vi "Main.vi"() -> ()   [LabVIEW 2018] (continued)
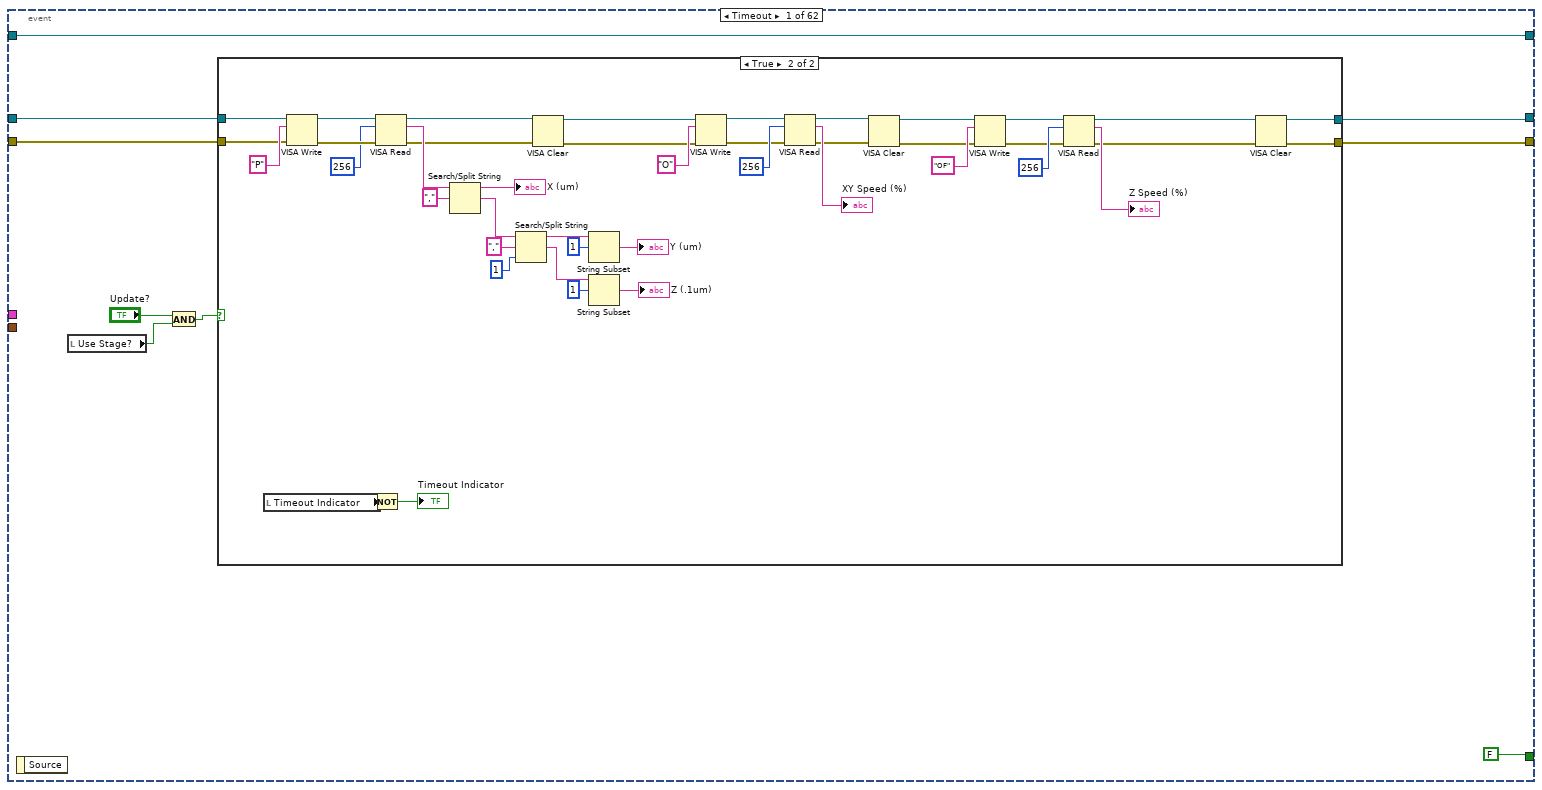
[diagram p4: hidden frame]
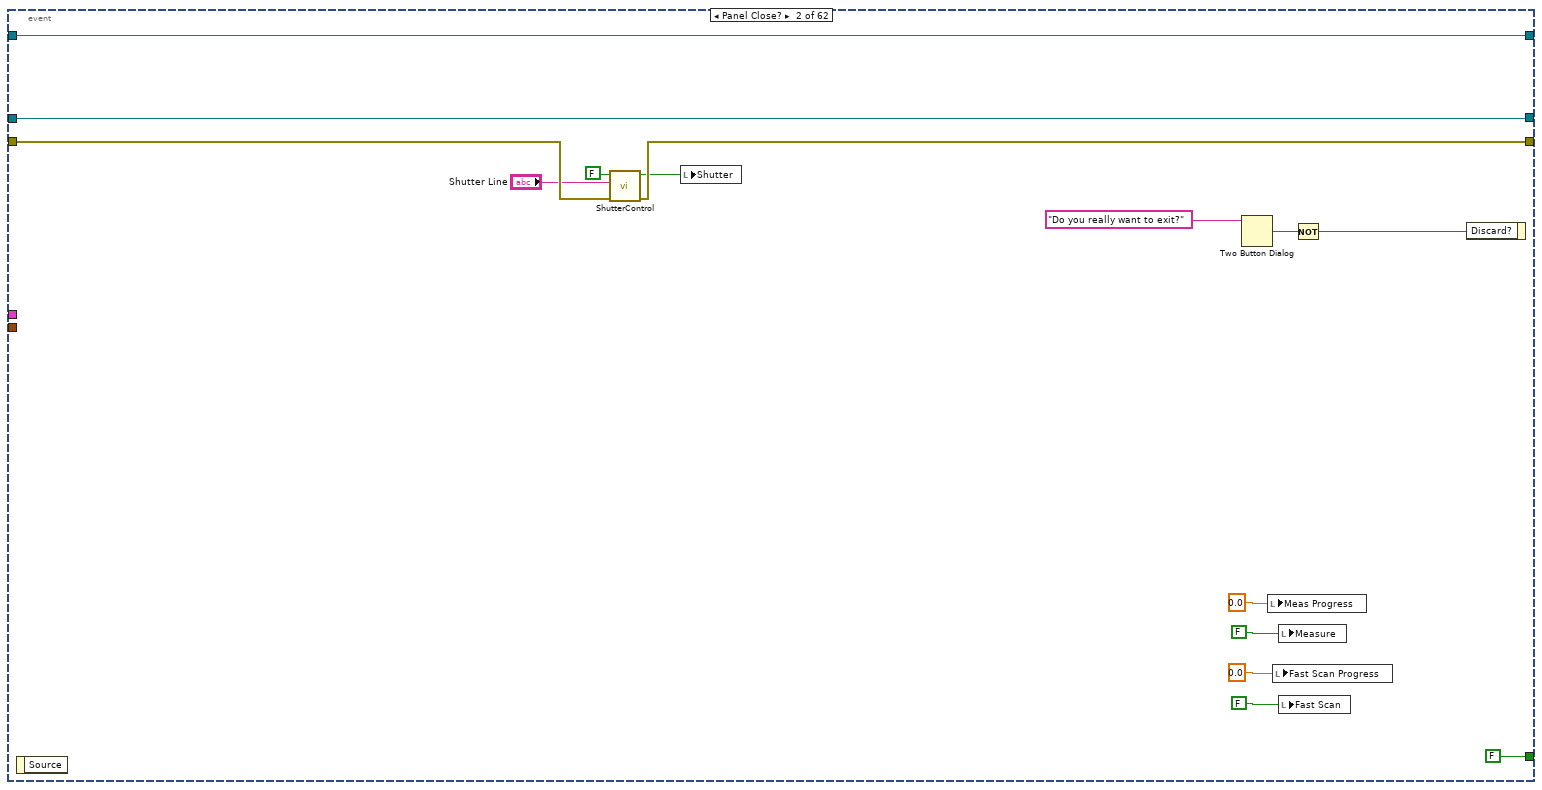
[diagram p6: hidden frame]
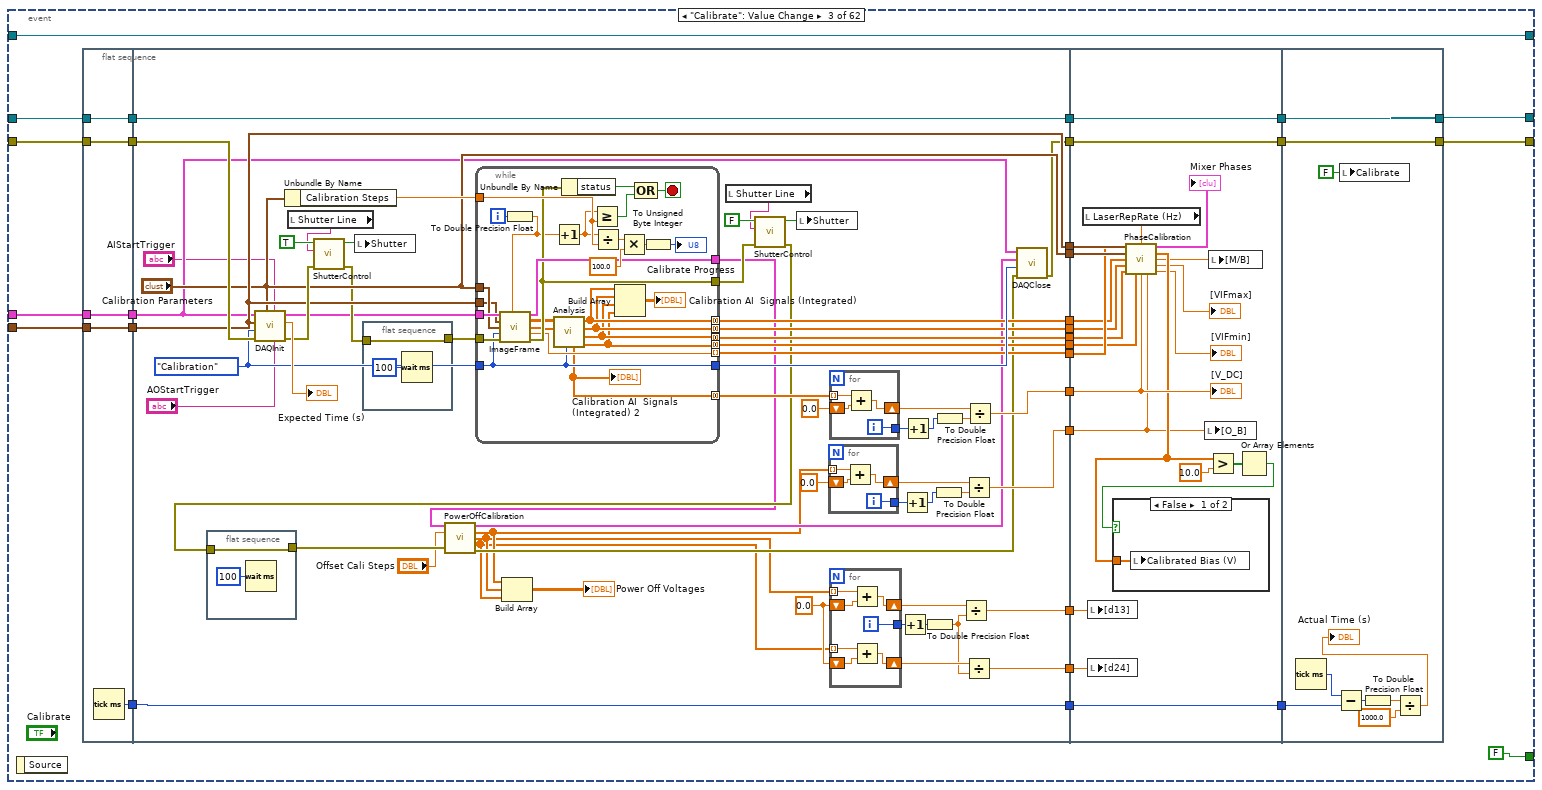
[diagram p7: hidden frame]
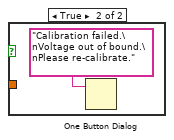
[diagram p8: hidden frame]
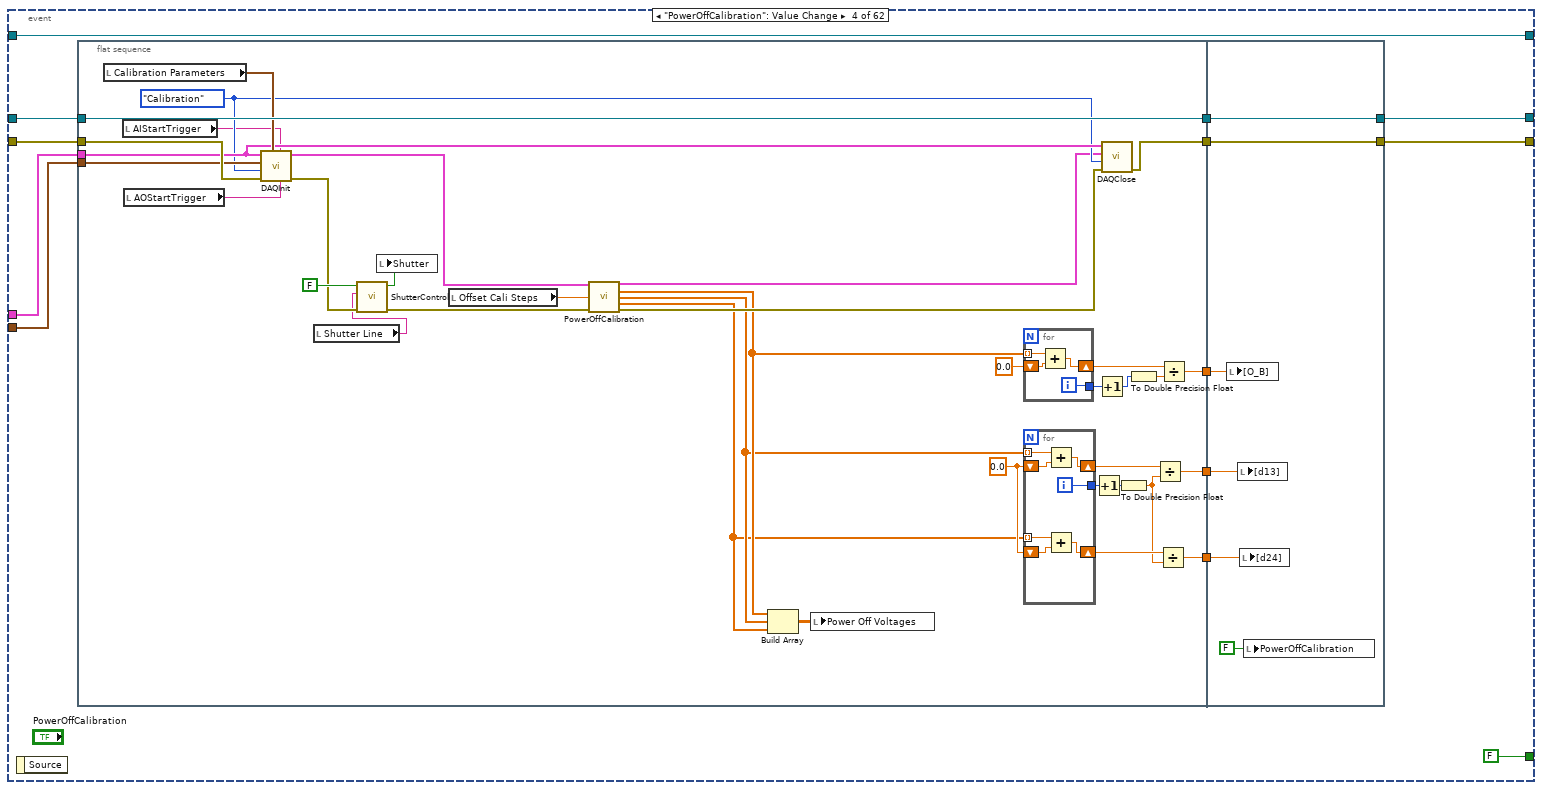
[diagram p9: hidden frame]
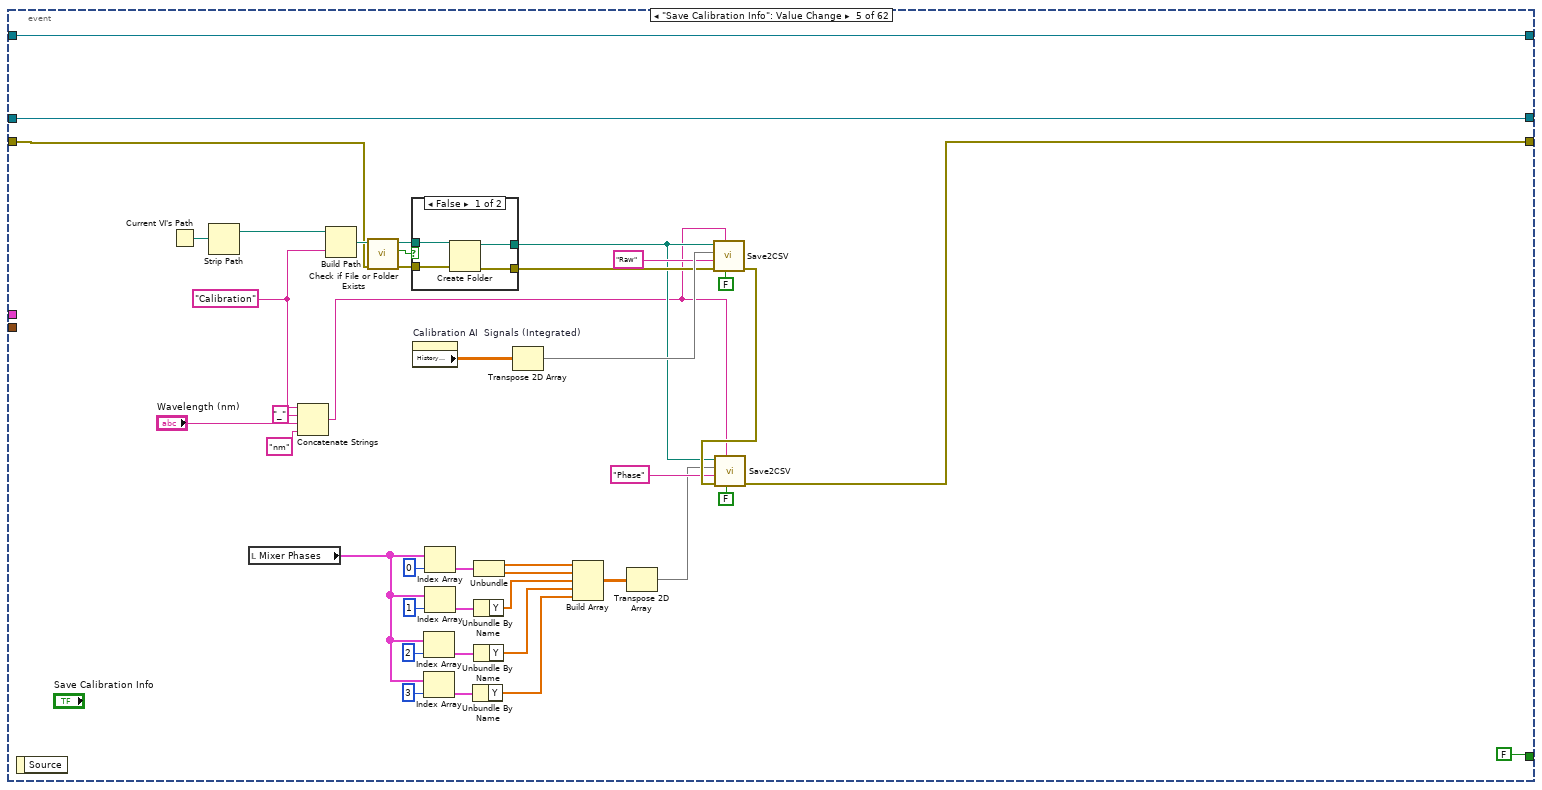
[diagram p10: hidden frame]
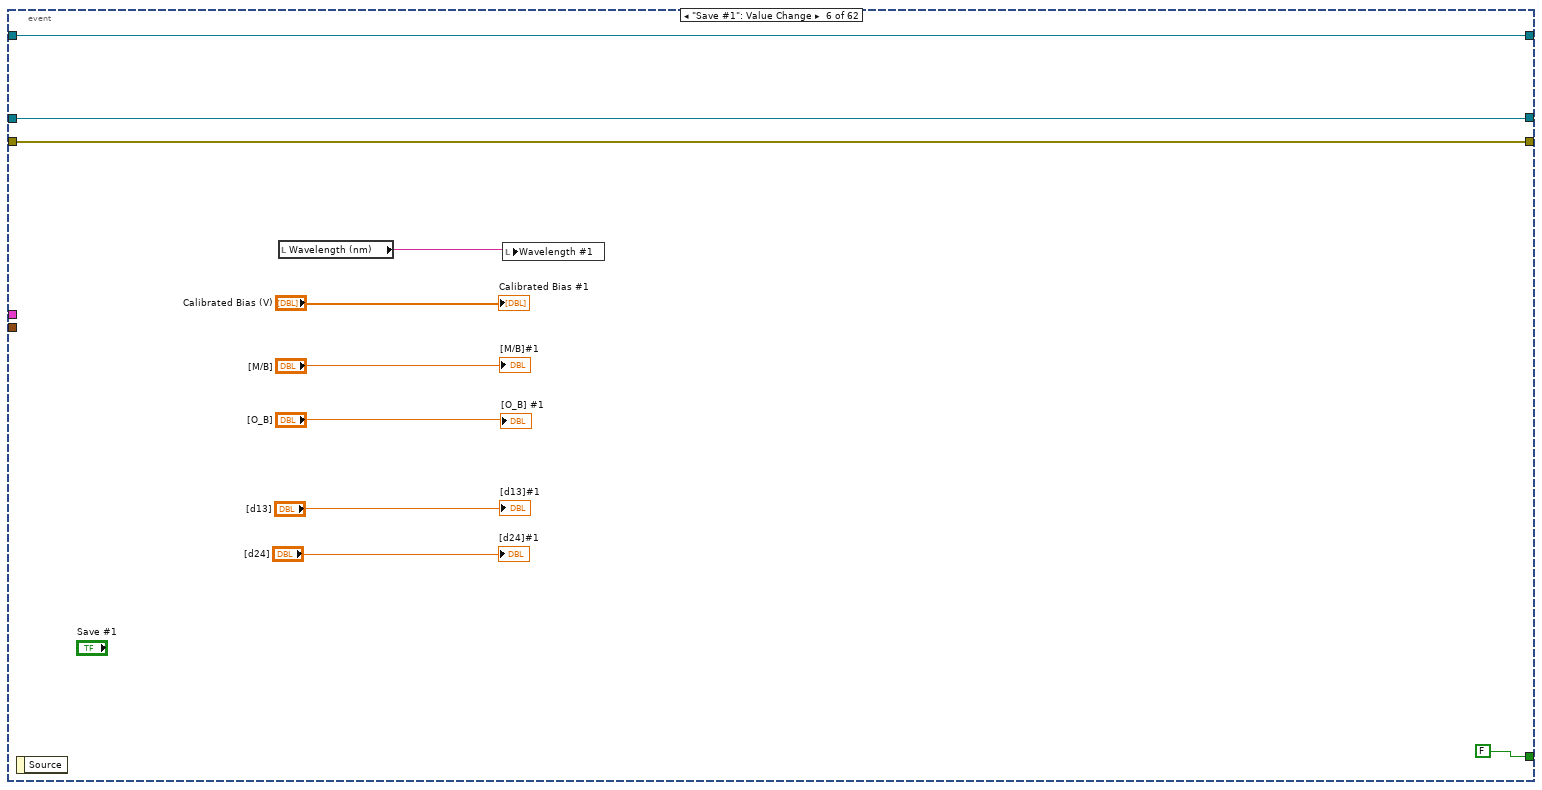
[diagram p12: hidden frame]
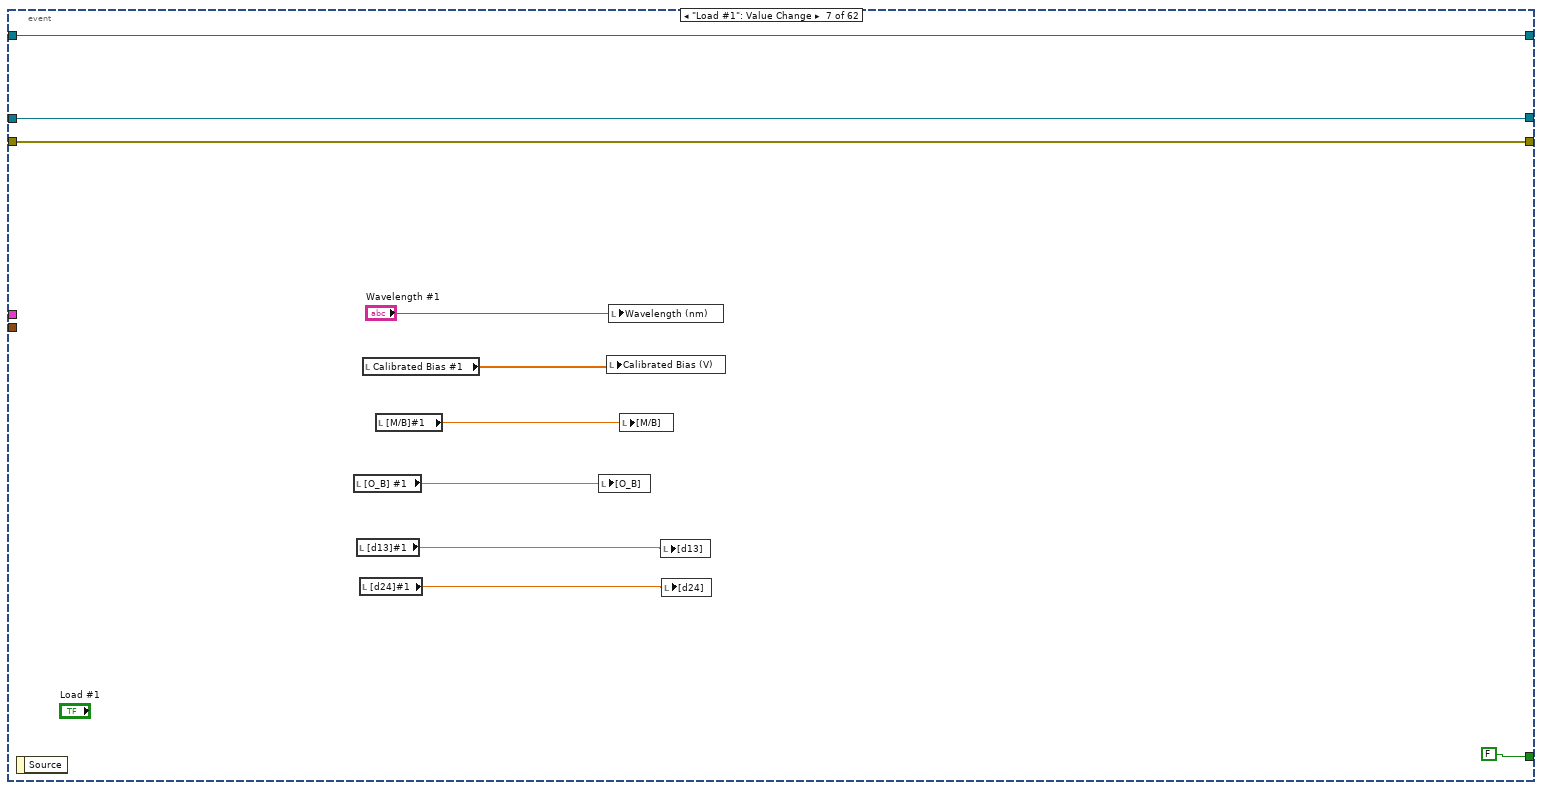
[diagram p13: hidden frame]
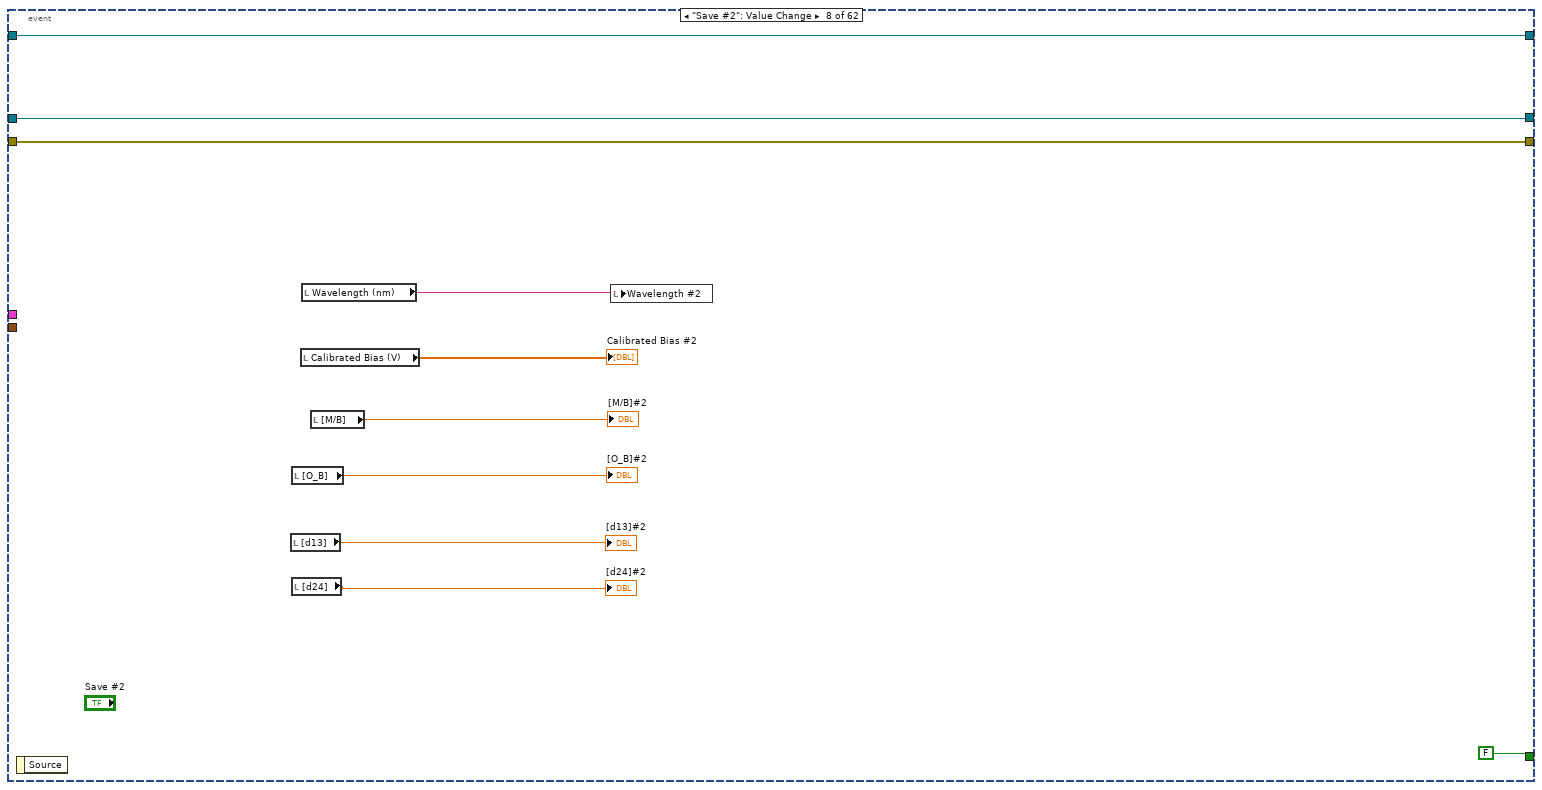
[diagram p14: hidden frame]
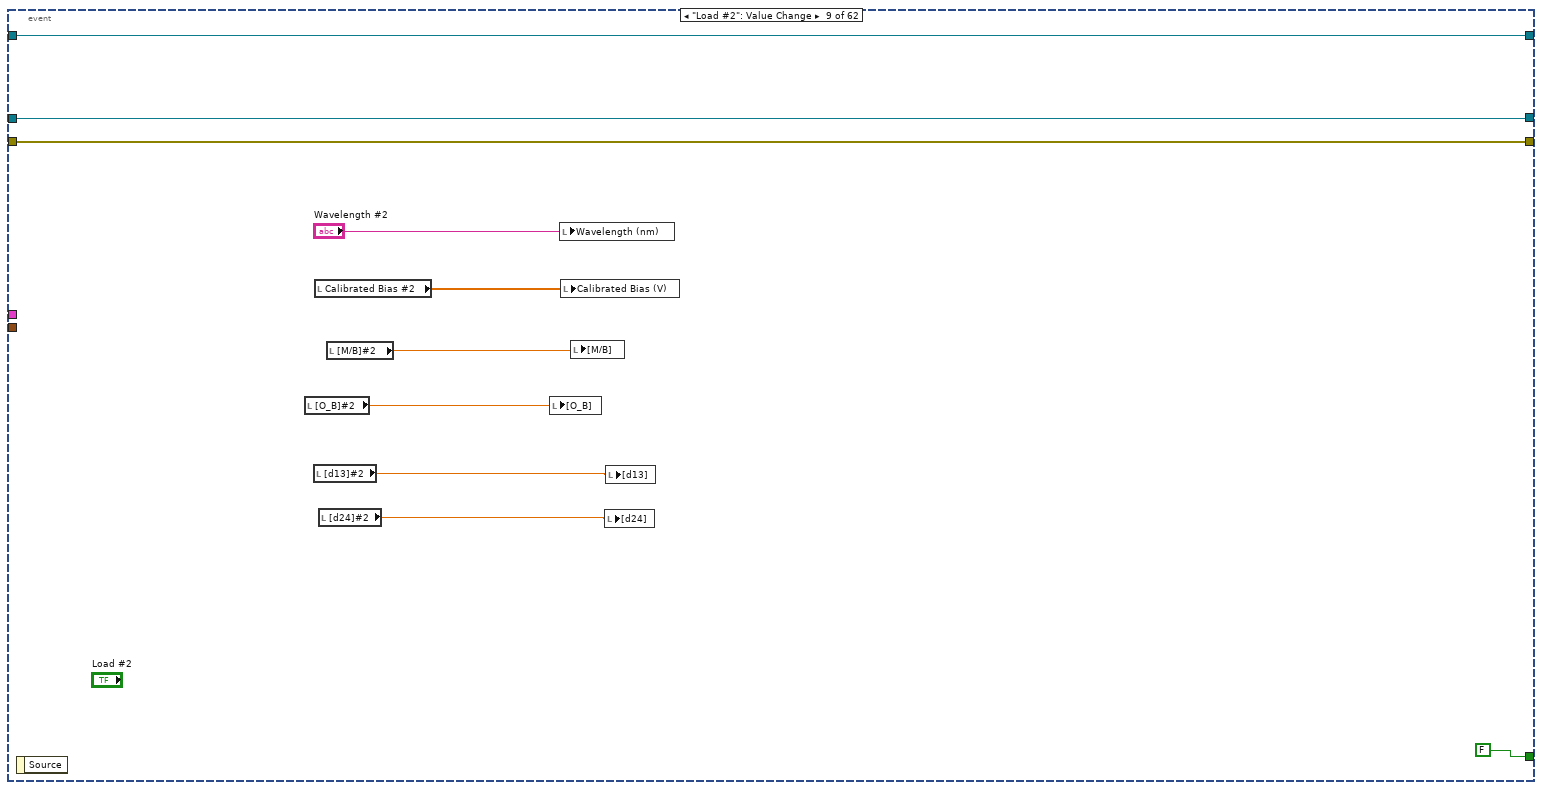
[diagram p15: hidden frame]
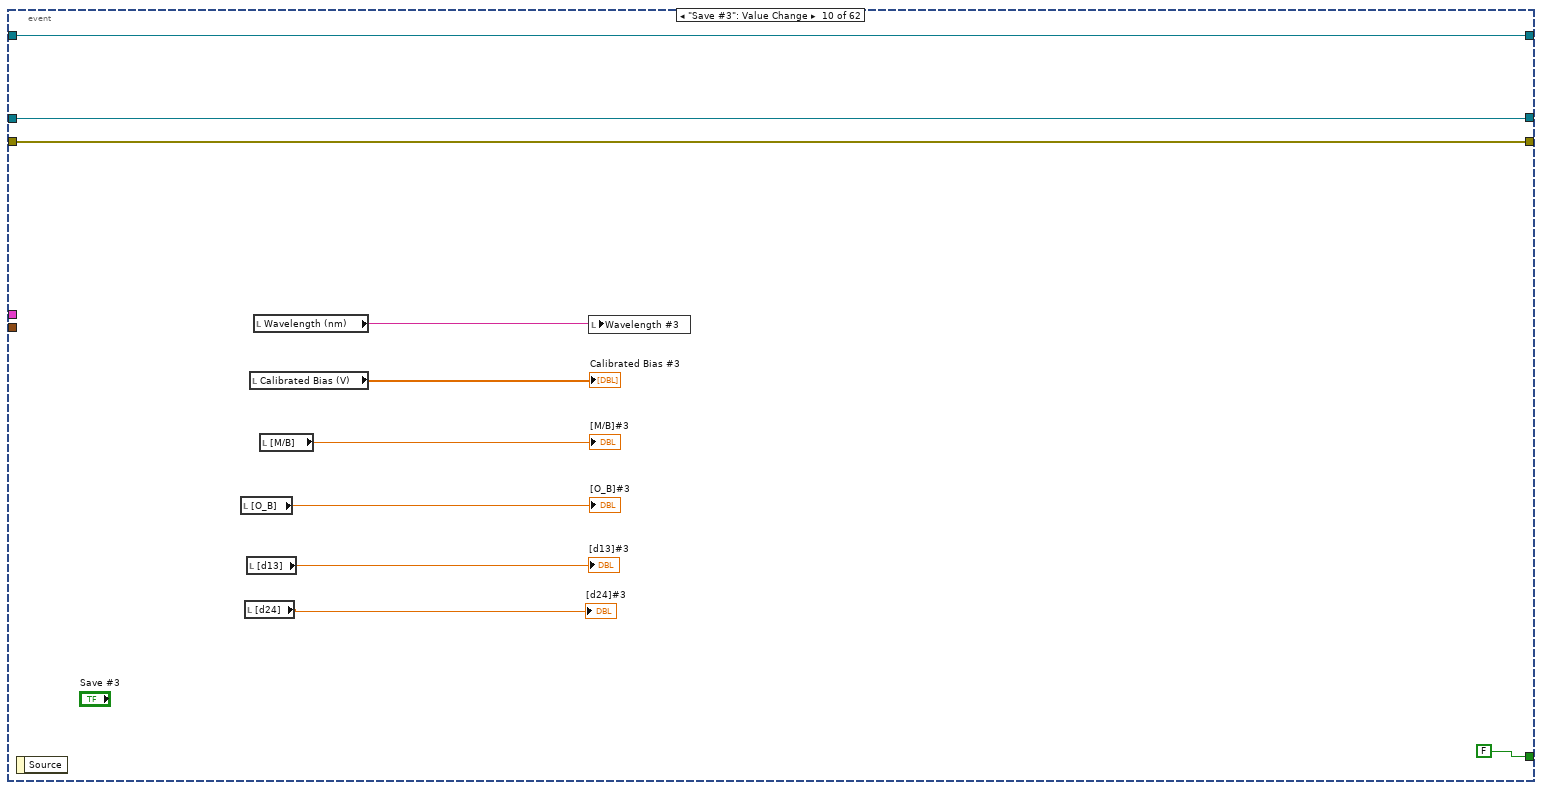
[diagram p16: hidden frame]
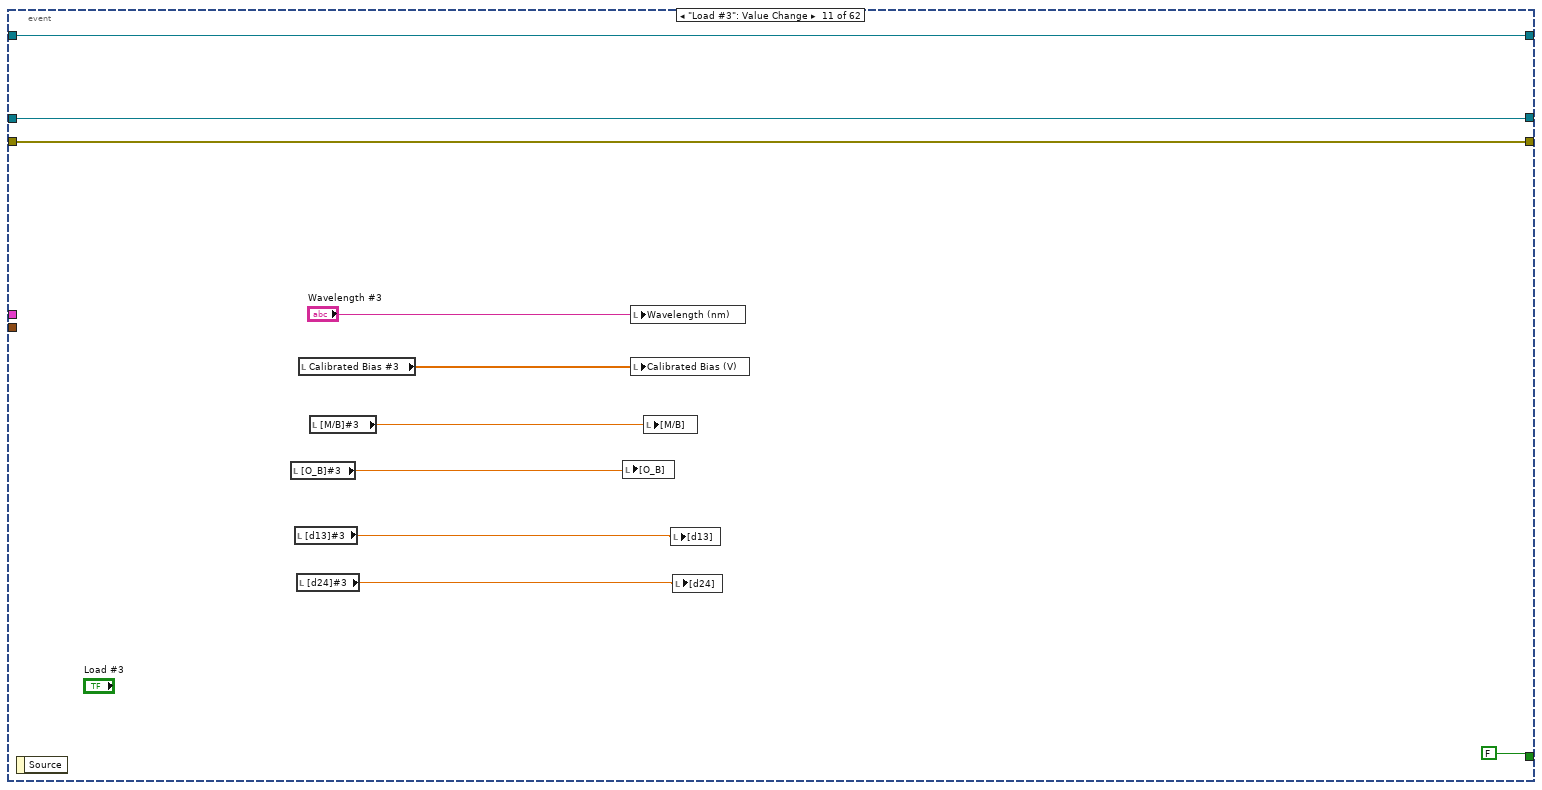
[diagram p17: hidden frame]
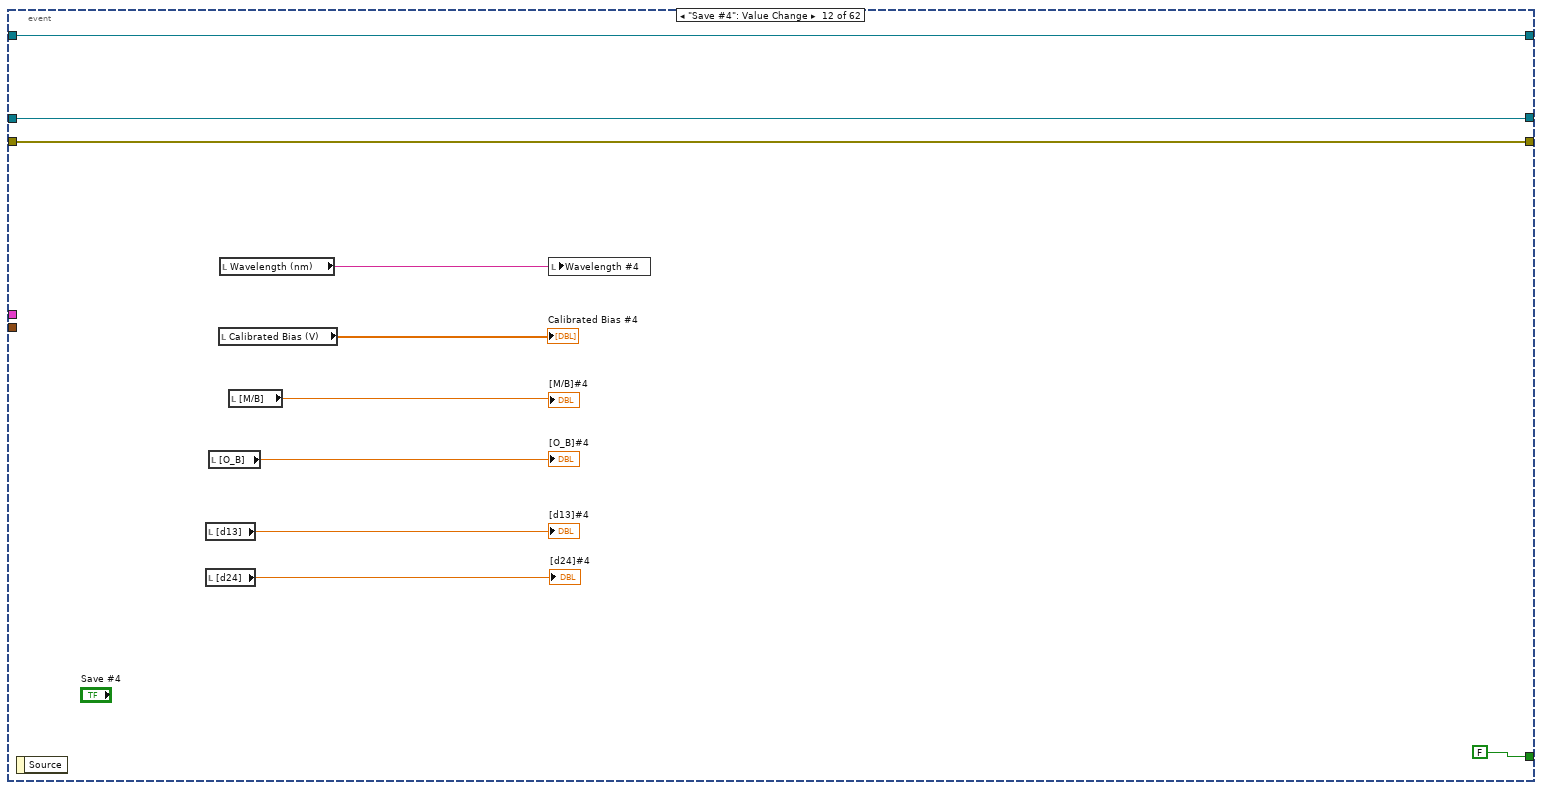
[diagram p18: hidden frame]
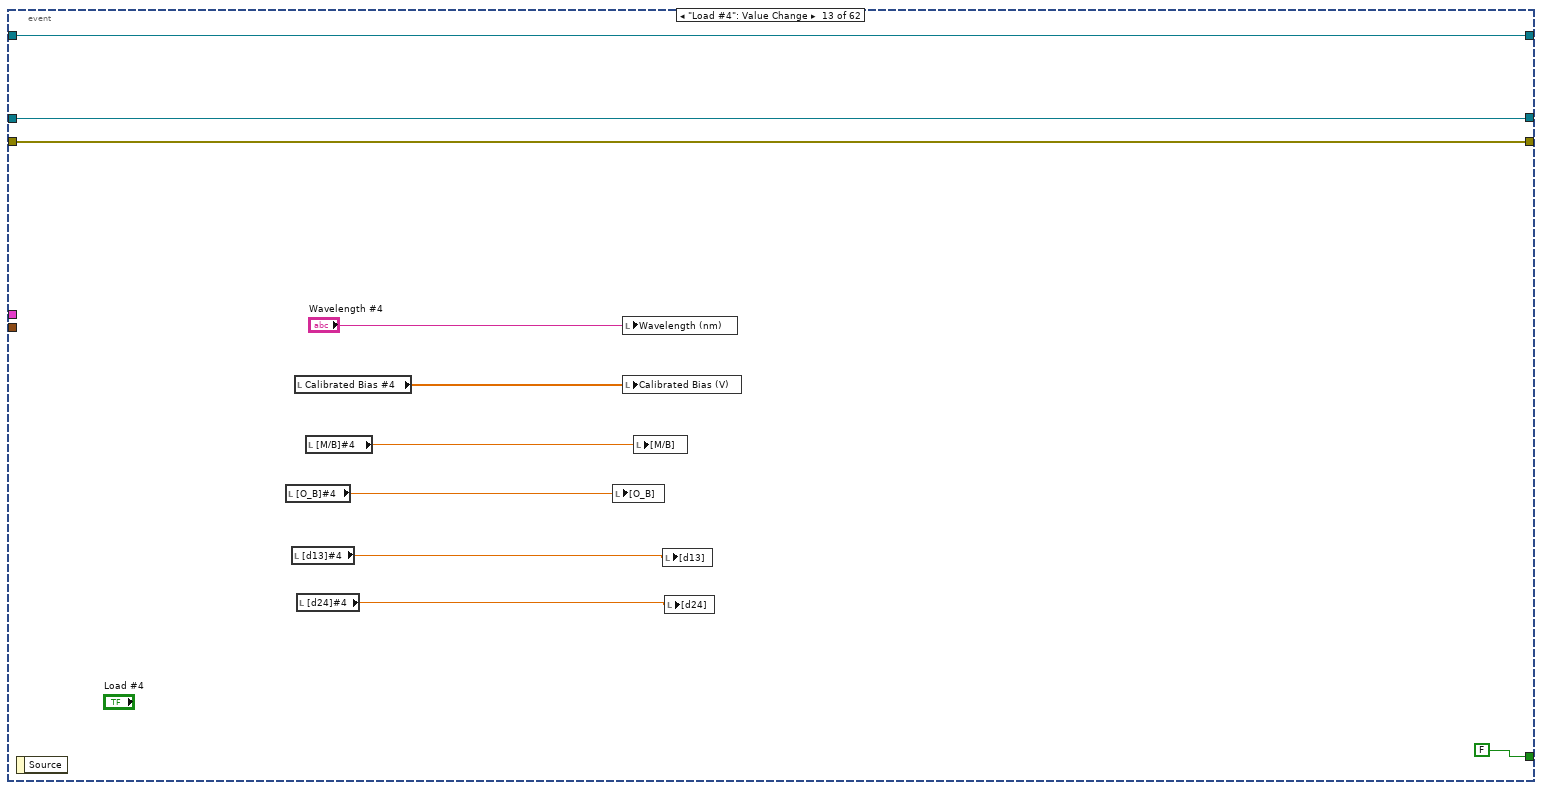
[diagram p19: hidden frame]
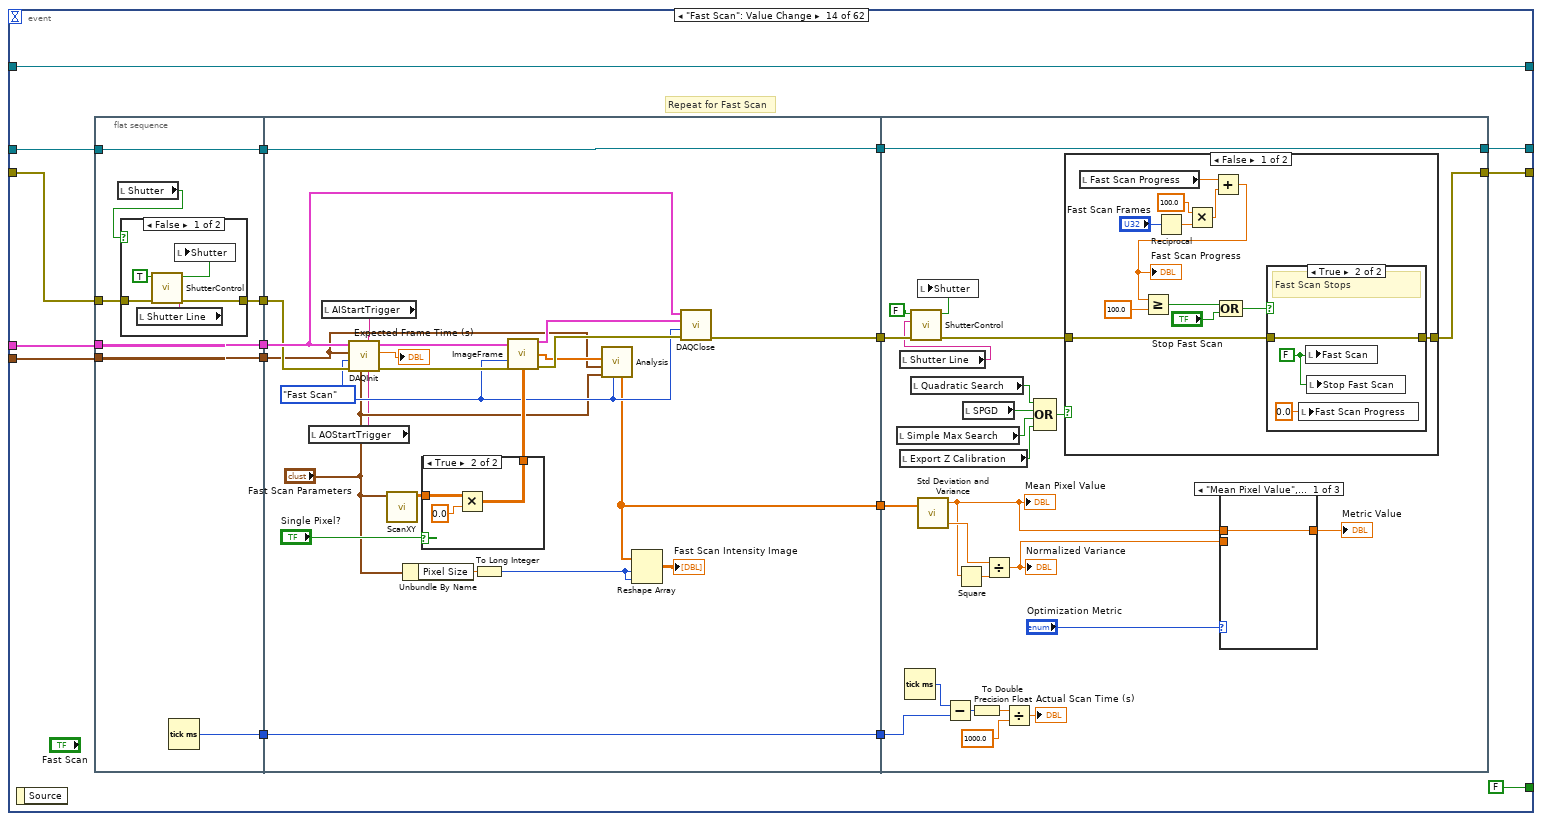
[diagram p20: hidden frame]
          }
        }
      }
      event "Set Current XY to 0": Value Change {
        n1487 = event-data() -> ()  [unwired: 1 in, 1 out]
        n1488 = local read "Use Stage?"() -> (w2774:bool)
        n1489 = case shown="True" w2774 {
          tunnel: w2780 -> [w2782 w2788]
          tunnel: w2779 -> [w2781 w2787]
          tunnel: [w2781 w2785] -> w2778
          tunnel: [w2782 w2784] -> w2777
          frame False {
          }
          frame True {
            n1490 = VISA Write(VISA resource name=w2788, write buffer="PS,0,0" ("string"), error in (no error)=w2787) -> (VISA resource name out=w2790:refnum<visa-resource-name>, error out=w2789:errorcluster)  [unwired: 1 out]
            n1491 = VISA Read(VISA resource name=w2790, byte count=u32 256, error in (no error)=w2789) -> (VISA resource name out=w2783:refnum<visa-resource-name>, error out=w2786:errorcluster)  [unwired: 2 out]
            n1492 = VISA Clear(VISA resource name=w2783, error in (no error)=w2786) -> (VISA resource name out=w2784:refnum<visa-resource-name>, error out=w2785:errorcluster)
          }
        }
      }
      event "Set Current Z to 0": Value Change {
        n1493 = event-data() -> ()  [unwired: 1 in, 1 out]
        n1494 = local read "Use Stage?"() -> (w2793:bool)
        n1495 = case shown="True" w2793 {
          tunnel: w2799 -> [w2801 w2807]
          tunnel: w2798 -> [w2800 w2806]
          tunnel: [w2800 w2804] -> w2797
          tunnel: [w2801 w2803] -> w2796
          frame False {
          }
          frame True {
            n1496 = VISA Write(VISA resource name=w2807, write buffer="PZ,0" ("string"), error in (no error)=w2806) -> (VISA resource name out=w2809:refnum<visa-resource-name>, error out=w2808:errorcluster)  [unwired: 1 out]
            n1497 = VISA Read(VISA resource name=w2809, byte count=u32 256, error in (no error)=w2808) -> (VISA resource name out=w2802:refnum<visa-resource-name>, error out=w2805:errorcluster)  [unwired: 2 out]
            n1498 = VISA Clear(VISA resource name=w2802, error in (no error)=w2805) -> (VISA resource name out=w2803:refnum<visa-resource-name>, error out=w2804:errorcluster)
          }
        }
      }
      event "Report Position": Value Change {
        n1499 = event-data() -> ()  [unwired: 1 in, 1 out]
        n1500 = local read "Use Stage?"() -> (w2812:bool)
        n1501 = case shown="True" w2812 {
          tunnel: w2818 -> [w2819 w2847]
          tunnel: w2817 -> [w2820 w2846]
          tunnel: [w2820 w2823] -> w2816
          tunnel: [w2819 w2822] -> w2815
          frame False {
          }
          frame True {
            n1502 = VISA Write(VISA resource name=w2846, write buffer="P" ("string"), error in (no error)=w2847) -> (VISA resource name out=w2853:refnum<visa-resource-name>, error out=w2852:errorcluster)  [unwired: 1 out]
            n1503 = VISA Read(VISA resource name=w2853, byte count=u32 256, error in (no error)=w2852) -> (VISA resource name out=w2829:refnum<visa-resource-name>, read buffer=w2858:string, error out=w2832:errorcluster)  [unwired: 1 out]
            n1504 = Search/Split String(string=w2858, search string/char (-)=",") -> (substring before match=w2845:string, match + rest of string=w2850:string)  [unwired: 1 in, 1 out]
            n1505 = Search/Split String(string=w2850, search string/char (-)=",", offset (0)=1) -> (substring before match=w2848:string, match + rest of string=w2859:string)  [unwired: 1 out]
            n1506 = local write "X (um)"(w2845) -> ()
            n1507 = String Subset(string=w2848, offset (0)=1) -> (substring=w2844:string)  [unwired: 1 in]
            n1508 = String Subset(string=w2859, offset (0)=1) -> (substring=w2843:string)  [unwired: 1 in]
            n1509 = VISA Clear(VISA resource name=w2829, error in (no error)=w2832) -> (VISA resource name out=w2830:refnum<visa-resource-name>, error out=w2831:errorcluster)
            n1510 = local write "Z (.1um)"(w2843) -> ()
            n1511 = local write "Y (um)"(w2844) -> ()
            n1512 = VISA Write(VISA resource name=w2830, write buffer="O" ("string"), error in (no error)=w2831) -> (VISA resource name out=w2840:refnum<visa-resource-name>, error out=w2841:errorcluster)  [unwired: 1 out]
            n1513 = VISA Read(VISA resource name=w2840, byte count=u32 256, error in (no error)=w2841) -> (VISA resource name out=w2828:refnum<visa-resource-name>, read buffer=w2834:string, error out=w2827:errorcluster)  [unwired: 1 out]
            n1514 = local write "XY Speed (%)"(w2834) -> ()
            n1515 = VISA Clear(VISA resource name=w2828, error in (no error)=w2827) -> (VISA resource name out=w2825:refnum<visa-resource-name>, error out=w2826:errorcluster)
            n1516 = VISA Write(VISA resource name=w2825, write buffer="OF" ("string"), error in (no error)=w2826) -> (VISA resource name out=w2836:refnum<visa-resource-name>, error out=w2837:errorcluster)  [unwired: 1 out]
            n1517 = VISA Read(VISA resource name=w2836, byte count=u32 256, error in (no error)=w2837) -> (VISA resource name out=w2824:refnum<visa-resource-name>, read buffer=w2833:string, error out=w2821:errorcluster)  [unwired: 1 out]
            n1518 = local write "Z Speed (%)"(w2833) -> ()
            n1519 = VISA Clear(VISA resource name=w2824, error in (no error)=w2821) -> (VISA resource name out=w2823:refnum<visa-resource-name>, error out=w2822:errorcluster)
          }
        }
      }
      event "Record X1": Value Change {
        n1520 = event-data() -> ()  [unwired: 1 in, 1 out]
        n1521 = property on="Fast Scan Intensity Image" class="IntGraph (strict)"(error in=w2864) -> (error out=w2863:errorcluster, "Cursor.Cursor X"=→"X1 (px)":dbl)  [unwired: 1 in, 1 out]
      }
      event "Record X2": Value Change {
        n1522 = event-data() -> ()  [unwired: 1 in, 1 out]
        n1523 = property on="Fast Scan Intensity Image" class="IntGraph (strict)"(error in=w2872) -> (error out=w2871:errorcluster, "Cursor.Cursor X"=→"X2 (px)":dbl)  [unwired: 1 in, 1 out]
      }
      event "Calculate Pixel Width": Value Change {
        n1524 = event-data() -> ()  [unwired: 1 in, 1 out]
        n1525 = local read "X2 (px)"() -> (w2878:dbl)
        n1526 = local read "X1 (px)"() -> (w2879:dbl)
        n1527 = Subtract(x=w2879, y=w2878) -> (x-y=w2880:dbl)
        n1528 = Absolute Value(x=w2880) -> (abs(x)=w2877:dbl)
        n1529 = Divide(x=30000.0, y=w2877) -> (x/y=→"dX (nm/px)":dbl)
      }
      event "Calculate XY Factor": Value Change {
        n1530 = event-data() -> ()  [unwired: 1 in, 1 out]
        n1531 = local read "Fast Scan Parameters"() -> (w2892:T4)
        n1532 = local read "dX (nm/px)"() -> (w2885:dbl)
        n1533 = Unbundle By Name(w2892) -> ("XY Factor (1/V)"=w2890:dbl)
        n1534 = Divide(x="Desired Pixel Width (nm)", y=w2885) -> (x/y=w2891:dbl)
        n1535 = Multiply(x=w2891, y=w2890) -> (x*y=→"New XY Factor":dbl)
      }
      event "Calculate XY Based on Objective": Value Change {
        # "XY Factor acquired at 400 pixel size, 300 nm pixel width"
        n1536 = event-data() -> ()  [unwired: 1 in, 1 out]
        n1537 = case shown="\"Nikon 40X NA 0.8 WD=3.5mm\", Default" "Objective Lens" {
          tunnel: [0.19061 ("x") 0.13615 ("x")] -> w2901
          frame "Nikon 40X NA 0.8 WD=3.5mm", Default {
          }
          frame "Olympus 25X NA 1.05 WD=2mm" {
          }
        }
        n1538 = local read "Fast Scan Parameters"() -> (w2904:T4)
        n1539 = local read "Desired Pixel Width (nm)"() -> (w2896:dbl)
        n1540 = Unbundle By Name(w2904) -> ("Pixel Size"=w2898:dbl)
        n1541 = Divide(x=w2898, y=400.0) -> (x/y=w2903:dbl)
        n1542 = Divide(x=w2896, y=300.0) -> (x/y=w2902:dbl)
        n1543 = Multiply(x=w2903, y=w2902) -> (x*y=w2900:dbl)
        n1544 = Multiply(x=w2901, y=w2900) -> (x*y=w2899:dbl)
        n1545 = local write "New XY Factor"(w2899) -> ()
      }
    }
  }
  n1546 = local read "Use Stage?"() -> (w1:bool)
  n1547 = case shown="True" w1 {
    tunnel: w19 -> [_ w2913]
    tunnel: w18 -> [w2910 w2912]
    tunnel: [w2910 w2911] -> w6
    frame False {
    }
    frame True {
      n1548 = VISA Close(VISA resource name=w2913, error in (no error)=w2912) -> (error out=w2911:errorcluster)
    }
  }
  n1549 = local read "Use DM?"() -> (w3:bool)
  n1550 = case shown="True" w3 {
    tunnel: w7 -> [_ w2917]
    tunnel: w6 -> [w2914 w2916]
    tunnel: [w2914 w2915] -> w5
    frame False {
    }
    frame True {
      n1551 = call "TLDFMX Close.vi"("error in (no error)"=w2916, "instrument handle"=w2917) -> ("error out"=w2915:errorcluster)  [unwired: 9 in]
    }
  }
  n1552 = call <vilib>:"Simple Error Handler.vi"("error in (no error)"=w5) -> ()  [unwired: 4 in, 5 out]
